vi "CRYO_MASTER_FULL_IP.vi"() -> ()   [LabVIEW 2017] (continued)
                n325 = invoke class="TabCtl (strict)" method="Get Image"(error in=errorcluster {"status"=FALSE, "code"=0, "source"=""} ("error in (no error)")) -> (error out=w580:errorcluster, "image data"=w582:T14)  [unwired: 5 in, 4 out]
                n326 = Build Path(base path=w591, name or relative path=w584) -> (appended path=w583:path)
                n327 = call <vilib>:"Write PNG File.vi"("error in (no error)"=w580, "image data"=w582, "path to PNG file"=w583) -> ("error out"=w578:errorcluster)  [unwired: 7 in, 1 out]
              }
            }
          }
          frame #1 {
            n328 = flat-sequence {
              tunnel: w595 -> [w598]
              tunnel: [w598] -> w594
              tunnel: w596 -> [w613]
              tunnel: w594 -> [w601]
              tunnel: [w600] -> w593
              tunnel: w592 -> [w599]
              frame #0 {
                n329 = property class="TabCtl (strict)"("Val(Sgnl)"=T2."LSI CONFIG" ("Value (Signaling)")) -> ()  [unwired: 2 in, 2 out]
              }
              frame #1 {
                w611 = "_" ("string")
                n330 = local read "Cycle #"() -> (w609:u32)
                n331 = call "LV_UNIXTIME.vi"("current time"=w601) -> ("date/time string"=w612:string)  [unwired: 9 in, 1 out]
                n332 = Format Value(format string="%06d", value (0)=w609) -> (output string=w608:string)  [unwired: 1 in]
                n333 = Concatenate Strings(w599, w612, w611, w608, w611, "page2.png" ("string")) -> (w606:string)
                n334 = invoke class="TabCtl (strict)" method="Get Image"(error in=errorcluster {"status"=FALSE, "code"=0, "source"=""} ("error in (no error)")) -> (error out=w602:errorcluster, "image data"=w604:T14)  [unwired: 5 in, 4 out]
                n335 = Build Path(base path=w613, name or relative path=w606) -> (appended path=w605:path)
                n336 = call <vilib>:"Write PNG File.vi"("error in (no error)"=w602, "image data"=w604, "path to PNG file"=w605) -> ("error out"=w600:errorcluster)  [unwired: 7 in, 1 out]
              }
            }
            n337 = local write "error out (frontpanel screenshots)"(w593) -> ()
          }
          frame #2 {
            n338 = flat-sequence {
              tunnel: w617 -> [w620]
              tunnel: [w620] -> w616
              tunnel: w618 -> [w635]
              tunnel: w616 -> [w623]
              tunnel: [w622] -> w615
              tunnel: w614 -> [w621]
              frame #0 {
                n339 = property class="TabCtl (strict)"("Val(Sgnl)"=T2."MEASUREMENT" ("Value (Signaling)")) -> ()  [unwired: 2 in, 2 out]
              }
              frame #1 {
                w633 = "_" ("string")
                n340 = local read "Cycle #"() -> (w631:u32)
                n341 = Format Value(format string="%06d", value (0)=w631) -> (output string=w630:string)  [unwired: 1 in]
                n342 = call "LV_UNIXTIME.vi"("current time"=w623) -> ("date/time string"=w634:string)  [unwired: 9 in, 1 out]
                n343 = Concatenate Strings(w621, w634, w633, w630, w633, "page3.png" ("string")) -> (w628:string)
                n344 = invoke class="TabCtl (strict)" method="Get Image"(error in=errorcluster {"status"=FALSE, "code"=0, "source"=""} ("error in (no error)")) -> (error out=w624:errorcluster, "image data"=w626:T14)  [unwired: 5 in, 4 out]
                n345 = Build Path(base path=w635, name or relative path=w628) -> (appended path=w627:path)
                n346 = call <vilib>:"Write PNG File.vi"("error in (no error)"=w624, "image data"=w626, "path to PNG file"=w627) -> ("error out"=w622:errorcluster)  [unwired: 7 in, 1 out]
              }
            }
            n347 = local write "error out (frontpanel screenshots)"(w615) -> ()
          }
          frame #3 {
            n348 = flat-sequence {
              tunnel: w639 -> [w642]
              tunnel: [w642] -> w638
              tunnel: w640 -> [w657]
              tunnel: w638 -> [w645]
              tunnel: [w644] -> w637
              tunnel: w636 -> [w643]
              frame #0 {
                n349 = property class="TabCtl (strict)"("Val(Sgnl)"=T2."HE AUTO FILL" ("Value (Signaling)")) -> ()  [unwired: 2 in, 2 out]
              }
              frame #1 {
                w655 = "_" ("string")
                n350 = local read "Cycle #"() -> (w653:u32)
                n351 = Format Value(format string="%06d", value (0)=w653) -> (output string=w652:string)  [unwired: 1 in]
                n352 = call "LV_UNIXTIME.vi"("current time"=w645) -> ("date/time string"=w656:string)  [unwired: 9 in, 1 out]
                n353 = Concatenate Strings(w643, w656, w655, w652, w655, "page4.png" ("string")) -> (w650:string)
                n354 = invoke class="TabCtl (strict)" method="Get Image"(error in=errorcluster {"status"=FALSE, "code"=0, "source"=""} ("error in (no error)")) -> (error out=w646:errorcluster, "image data"=w648:T14)  [unwired: 5 in, 4 out]
                n355 = Build Path(base path=w657, name or relative path=w650) -> (appended path=w649:path)
                n356 = call <vilib>:"Write PNG File.vi"("error in (no error)"=w646, "image data"=w648, "path to PNG file"=w649) -> ("error out"=w644:errorcluster)  [unwired: 7 in, 1 out]
              }
            }
            n357 = local write "error out (frontpanel screenshots)"(w637) -> ()
          }
          frame #4 {
            n358 = flat-sequence {
              tunnel: w661 -> [w664]
              tunnel: [w664] -> w660
              tunnel: w662 -> [w679]
              tunnel: w660 -> [w667]
              tunnel: [w666] -> w659
              tunnel: w658 -> [w665]
              frame #0 {
                n359 = property class="TabCtl (strict)"("Val(Sgnl)"=T2."VALVE/HEATER CTRL" ("Value (Signaling)")) -> ()  [unwired: 2 in, 2 out]
              }
              frame #1 {
                w677 = "_" ("string")
                n360 = local read "Cycle #"() -> (w675:u32)
                n361 = call "LV_UNIXTIME.vi"("current time"=w667) -> ("date/time string"=w678:string)  [unwired: 9 in, 1 out]
                n362 = Format Value(format string="%06d", value (0)=w675) -> (output string=w674:string)  [unwired: 1 in]
                n363 = Concatenate Strings(w665, w678, w677, w674, w677, "page5.png" ("string")) -> (w672:string)
                n364 = invoke class="TabCtl (strict)" method="Get Image"(error in=errorcluster {"status"=FALSE, "code"=0, "source"=""} ("error in (no error)")) -> (error out=w668:errorcluster, "image data"=w670:T14)  [unwired: 5 in, 4 out]
                n365 = Build Path(base path=w679, name or relative path=w672) -> (appended path=w671:path)
                n366 = call <vilib>:"Write PNG File.vi"("error in (no error)"=w668, "image data"=w670, "path to PNG file"=w671) -> ("error out"=w666:errorcluster)  [unwired: 7 in, 1 out]
              }
            }
            n367 = local write "error out (frontpanel screenshots)"(w659) -> ()
          }
          frame #5 {
            n368 = flat-sequence {
              tunnel: w683 -> [w686]
              tunnel: [w686] -> w682
              tunnel: w684 -> [w701]
              tunnel: w682 -> [w689]
              tunnel: [w688] -> w681
              tunnel: w680 -> [w687]
              frame #0 {
                n369 = property class="TabCtl (strict)"("Val(Sgnl)"=T2."DMMs" ("Value (Signaling)")) -> ()  [unwired: 2 in, 2 out]
              }
              frame #1 {
                w699 = "_" ("string")
                n370 = local read "Cycle #"() -> (w697:u32)
                n371 = call "LV_UNIXTIME.vi"("current time"=w689) -> ("date/time string"=w700:string)  [unwired: 9 in, 1 out]
                n372 = Format Value(format string="%06d", value (0)=w697) -> (output string=w696:string)  [unwired: 1 in]
                n373 = Concatenate Strings(w687, w700, w699, w696, w699, "page6.png" ("string")) -> (w694:string)
                n374 = invoke class="TabCtl (strict)" method="Get Image"(error in=errorcluster {"status"=FALSE, "code"=0, "source"=""} ("error in (no error)")) -> (error out=w690:errorcluster, "image data"=w692:T14)  [unwired: 5 in, 4 out]
                n375 = Build Path(base path=w701, name or relative path=w694) -> (appended path=w693:path)
                n376 = call <vilib>:"Write PNG File.vi"("error in (no error)"=w690, "image data"=w692, "path to PNG file"=w693) -> ("error out"=w688:errorcluster)  [unwired: 7 in, 1 out]
              }
            }
            n377 = local write "error out (frontpanel screenshots)"(w681) -> ()
          }
          frame #6 {
            n378 = flat-sequence {
              tunnel: w705 -> [w708]
              tunnel: [w708] -> w704
              tunnel: w706 -> [w723]
              tunnel: w704 -> [w711]
              tunnel: [w710] -> w703
              tunnel: w702 -> [w709]
              frame #0 {
                n379 = property class="TabCtl (strict)"("Val(Sgnl)"=T2."DIAGRAM" ("Value (Signaling)")) -> ()  [unwired: 2 in, 2 out]
              }
              frame #1 {
                w721 = "_" ("string")
                n380 = local read "Cycle #"() -> (w719:u32)
                n381 = Format Value(format string="%06d", value (0)=w719) -> (output string=w718:string)  [unwired: 1 in]
                n382 = call "LV_UNIXTIME.vi"("current time"=w711) -> ("date/time string"=w722:string)  [unwired: 9 in, 1 out]
                n383 = Concatenate Strings(w709, w722, w721, w718, w721, "page7.png" ("string")) -> (w716:string)
                n384 = invoke class="TabCtl (strict)" method="Get Image"(error in=errorcluster {"status"=FALSE, "code"=0, "source"=""} ("error in (no error)")) -> (error out=w712:errorcluster, "image data"=w714:T14)  [unwired: 5 in, 4 out]
                n385 = Build Path(base path=w723, name or relative path=w716) -> (appended path=w715:path)
                n386 = call <vilib>:"Write PNG File.vi"("error in (no error)"=w712, "image data"=w714, "path to PNG file"=w715) -> ("error out"=w710:errorcluster)  [unwired: 7 in, 1 out]
              }
            }
            n387 = local write "error out (frontpanel screenshots)"(w703) -> ()
          }
          frame #7 {
            n388 = flat-sequence {
              tunnel: w727 -> [w730]
              tunnel: [w730] -> w726
              tunnel: w728 -> [w745]
              tunnel: w726 -> [w733]
              tunnel: [w732] -> w725
              tunnel: w724 -> [w731]
              frame #0 {
                n389 = property class="TabCtl (strict)"("Val(Sgnl)"=T2."(Plc. hld.)" ("Value (Signaling)")) -> ()  [unwired: 2 in, 2 out]
              }
              frame #1 {
                w743 = "_" ("string")
                n390 = local read "Cycle #"() -> (w741:u32)
                n391 = Format Value(format string="%06d", value (0)=w741) -> (output string=w740:string)  [unwired: 1 in]
                n392 = call "LV_UNIXTIME.vi"("current time"=w733) -> ("date/time string"=w744:string)  [unwired: 9 in, 1 out]
                n393 = Concatenate Strings(w731, w744, w743, w740, w743, "page8.png" ("string")) -> (w738:string)
                n394 = invoke class="TabCtl (strict)" method="Get Image"(error in=errorcluster {"status"=FALSE, "code"=0, "source"=""} ("error in (no error)")) -> (error out=w734:errorcluster, "image data"=w736:T14)  [unwired: 5 in, 4 out]
                n395 = Build Path(base path=w745, name or relative path=w738) -> (appended path=w737:path)
                n396 = call <vilib>:"Write PNG File.vi"("error in (no error)"=w734, "image data"=w736, "path to PNG file"=w737) -> ("error out"=w732:errorcluster)  [unwired: 7 in, 1 out]
              }
            }
            n397 = local write "error out (frontpanel screenshots)"(w725) -> ()
          }
          frame #8 {
            n398 = local write "Frontpanel screenshots"(FALSE ("Frontpanel screenshots")) -> ()
          }
        }
        "error out (frontpanel screenshots)" <- w566
        n399 = property class="TabCtl (strict)"("Val(Sgnl)"=w564) -> ()  [unwired: 2 in, 2 out]
      }
      event "Stop Button": Value Change {
        n400 = event-data() -> ()  [unwired: 1 in, 3 out]
      }
    }
    n401 = Wait (ms)(milliseconds to wait=u32 123) -> ()  [unwired: 1 out]
  }
  n402 = while {
    stop <- w748 stop-if-true
    n403 = Wait (ms)(milliseconds to wait=u32 101) -> ()  [unwired: 1 out]
    n404 = event shown="[2] Timeout" {
      selector: _ -> [_ _ _]
      dyn-events: _ -> [_ _ _]
      timeout: _ -> [_ _ _]
      tunnel: [FALSE TRUE FALSE] -> w748
      event "Initialize (DMMs)": Value Change {
        w751 = T1 [] ("Value (Signaling)")
        n405 = event-data() -> ()  [unwired: 1 in, 3 out]
        n406 = property on="Graph DMMs 1" class="XYGraph (strict)"("Val(Sgnl)"=w751) -> ()  [unwired: 2 in, 2 out]
        n407 = property on="Graph DMMs 2" class="XYGraph (strict)"("Val(Sgnl)"=w751) -> ()  [unwired: 2 in, 2 out]
      }
      event "Stop Button": Value Change {
        n408 = event-data() -> ()  [unwired: 1 in, 3 out]
      }
      event Timeout {
        n409 = event-data() -> ()  [unwired: 1 in, 3 out]
      }
    }
  }
  n410 = Obtain Notifier(name (unnamed)="stop notifier", notification data type=w9, create if not found? (T)=w9, error in (no error)=errorcluster {"status"=FALSE, "code"=0, "source"=""}) -> (notifier out=w3:refnum<notifier>, error out=w2:errorcluster)  [unwired: 1 out]
  n411 = while {
    shift-right: [w852] -> w36
    shift-left: refnum<class "USBData.lvclass"> refnum ("USBData.lvclass") -> [w855]
    shift-right: [w848] -> w35
    shift-left: errorcluster {"status"=FALSE, "code"=0, "source"=""} ("error in (no error)") -> [w854]
    tunnel: "RUN label" -> [w760]
    tunnel: "Base Path" -> [w792]
    shift-right: [w830] -> w29
    shift-left: errorcluster {"status"=FALSE, "code"=0, "source"=""} ("error in (no error)") -> [w846]
    shift-right: [w831] -> w30
    shift-left: refnum<class "LSI218Data.lvclass"> refnum ("LSI218Data.lvclass") -> [w845]
    shift-right: [w818] -> w26
    shift-left: refnum<class "LSI336Data.lvclass"> refnum ("LSI336Data.lvclass") -> [w827]
    shift-right: [w817] -> w25
    shift-left: w15 -> [w826]
    shift-right: [w806] -> _
    shift-left: errorcluster {"status"=FALSE, "code"=0, "source"=""} ("error in") -> [w807]
    shift-right: [w796] -> w19
    shift-left: refnum<class "USBData.lvclass"> refnum ("USBData.lvclass") -> [w804]
    shift-right: [w795] -> w18
    shift-left: errorcluster {"status"=FALSE, "code"=0, "source"=""} ("error in (no error)") -> [w803]
    shift-right: [w791] -> _
    shift-left: w15 -> [w790]
    tunnel: w3 -> [w758]
    tunnel: w2 -> [w757]
    tunnel: [w755] -> w5
    tunnel: [w754] -> w4
    i -> [w767]
    stop <- "Stop Button" stop-if-true
    w813 = u32 24 ("Number of Rows")
    w823 = T20 [] ("appended array")
    w840 = T20 [] ("appended array")
    n412 = local read "LSI218Settings(A-F)"() -> (w782:T4)
    n413 = control-ref of="Plot selecter LSI218(2)\n    1      2     3     4"() -> (w811:refnum<vi>)
    n414 = control-ref of="Plot selecter LSI218(1)\n    1      2     3     4"() -> (w812:refnum<vi>)
    n415 = control-ref of="Plot selecter LSI336 \n     1      2     3     4"() -> (w810:refnum<vi>)
    n416 = property on="Property Node" class="Arr (strict)"(reference=w811, "Number of Rows"=w813) -> ()  [unwired: 1 in, 2 out]
    n417 = property on="Property Node" class="Arr (strict)"(reference=w812, "Number of Rows"=w813) -> ()  [unwired: 1 in, 2 out]
    n418 = local read "LSI336Settings(X,Y)"() -> (w780:T4)
    n419 = Array Size(array=w782) -> (size(s)=w781:i32)
    n420 = property on="Property Node" class="Arr (strict)"(reference=w810, "Number of Rows"=u32 8) -> ()  [unwired: 1 in, 2 out]
    n421 = Multiply(x="Measurement Interval (s)", y=u32 1000) -> (x*y=w849:dbl)
    n422 = Wait (ms)(milliseconds to wait=w849) -> ()  [unwired: 1 out]
    n423 = for {
      N: w781 -> [_]
      tunnel: w782 -> [w866] mode=indexing
      tunnel: [w865] -> w778 mode=concatenating
      n424 = Unbundle By Name(w866) -> ("SensorLocations"=w865:T13)
    }
    n425 = for {
      tunnel: w780 -> [w864] mode=indexing
      tunnel: [w863] -> w779 mode=concatenating
      n426 = Unbundle By Name(w864) -> ("SensorLocations"=w863:T13)
    }
    n427 = Quotient & Remainder(x=w767, y="Screenshots interval") -> (x-y*floor(x/y)=w765:i64)  [unwired: 1 out]
    n428 = Equal?(x=w767, y=0) -> (x = y?=w759:bool)
    n429 = case shown="True" w759 {
      tunnel: w855 -> [w1904 w1927]
      tunnel: w854 -> [w1898 w1925]
      tunnel: w767 -> [w1889 _]
      tunnel: [w1896 w1922] -> w848
      tunnel: [w1893 w1921] -> w805
      tunnel: [w1894 w1920] -> w852
      tunnel: [w1884 w1915] -> w853
      tunnel: w792 -> [_ w1914]
      tunnel: [w1883 w1911] -> w787
      frame False {
        n430 = call-dynamic "USBData_measure.vi"("USBData in"=w1904, "DAQ sample #"=i64 5, "DAQ timeout"=100.0 ("DAQ timeout (def: 100)"), "MeasurementIndex"=w1889, "error in (no error)"=w1898, "save every ... measurements"="Record interval") -> ("USBData out"=w1903:refnum<class "USBData.lvclass">, "TimeMeasuremeent"=w1900:timestamp, "Status"=→"USB6210 Status":T6, "LastDataAcquired"=w1885:dbl[], "error out"=w1899:errorcluster)  [unwired: 3 in, 2 out]
        "Time of Last Measurement (USB6210)" <- w1900
        "Last Vol\n(USB6210)" <- w1885
        n431 = call-dynamic "USBData_convert.vi"("Save every ... measurements"="Record interval", "MeasurementIndex"=w1889, "error in (no error)"=w1899, "LastDataAcquired"=w1885, "TimeMeasuremeent"=w1900, "USBData in"=w1903) -> ("error out"=w1897:errorcluster, "LeakDet_FULL"=w1892:dbl, "LastDataConverted"=w1886:dbl[], "USBData out"=w1895:refnum<class "USBData.lvclass">)  [unwired: 2 in]
        n432 = call "USBData_read.vi"("USBData in"=w1895, "error in (no error)"=w1897) -> ("Status"=w1887:T6, "USBData out"=w1894:refnum<class "USBData.lvclass">, "Data"=w1893:T21, "Basic"=w1884:T22, "error out"=w1896:errorcluster)  [unwired: 2 in, 2 out]
        n433 = local write "USB6210 Status"(w1887) -> ()
        n434 = Unbundle By Name(w1884) -> ("ReadLeakDet?"=w1891:bool)
        n435 = Unbundle By Name(w1884) -> ("Labels"=w1883:string[])
        n436 = case shown="False" w1891 {
          tunnel: w1886 -> [w1905 w1908]
          tunnel: w1892 -> [_ w1907]
          tunnel: [w1905 w1906] -> w1890
          frame False {
          }
          frame True {
            n437 = Build Array (concatenate)(w1908, w1907) -> (w1906:dbl[])
          }
        }
        "Last Data \n(USB6210)" <- w1890
      }
      frame True {
        n438 = local read "RUN Identifier"() -> (w1909:string)
        n439 = call-dynamic "USBData_initialize.vi"("USBData in"=w1927, "SeriesSetting"="USB6210 Config", "BasePath"=w1914, "RunIdentifier"=w1909, "FileName"="InstName (USB6210)", "error in (no error)"=w1925) -> ("Status"=w1910:T6, "USBData out"=w1923:refnum<class "USBData.lvclass">, "error out"=w1924:errorcluster)  [unwired: 5 in, 2 out]
        n440 = local write "USB6210 Status"(w1910) -> ()
        n441 = call "USBData_read.vi"("USBData in"=w1923, "error in (no error)"=w1924) -> ("Status"=w1913:T6, "USBData out"=w1920:refnum<class "USBData.lvclass">, "Data"=w1921:T21, "Basic"=w1915:T22, "error out"=w1922:errorcluster)  [unwired: 2 in, 2 out]
        n442 = local write "USB6210 Status"(w1913) -> ()
        n443 = Unbundle By Name(w1915) -> ("ReadLeakDet?"=w1919:bool, "Labels"=w1911:string[])
        n444 = Array Size(array=w1911) -> (size(s)=w1918:i32)
        n445 = case shown="True" w1919 {
          tunnel: w1918 -> [w1928 w1930]
          tunnel: [w1928 w1929] -> w1916
          frame False {
          }
          frame True {
            n446 = Add(x=w1930, y=1) -> (x+y=w1929:i32)
          }
        }
        n447 = Initialize Array(TRUE ("Activate 2"), w1916) -> ()  [unwired: 1 out]
      }
    }
    "error out (USB6210)" <- w848
    n448 = case shown="False" w759 {
      tunnel: [w1437 w1464] -> w795
      tunnel: [w1434 w1463] -> w802
      tunnel: [w1435 w1462] -> w796
      tunnel: [w1426 w1457] -> w801
      tunnel: [w1425 w1455] -> _
      tunnel: w804 -> [w1424 w1453]
      tunnel: w792 -> [_ w1452]
      tunnel: w803 -> [w1423 w1451]
      tunnel: w767 -> [w1422 _]
      frame False {
        n449 = local read "Record interval"() -> (w1421:i64)
        n450 = call-dynamic "USBData_measure.vi"("USBData in"=w1424, "DAQ sample #"=i64 5, "DAQ timeout"=100.0 ("DAQ timeout (def: 100)"), "MeasurementIndex"=w1422, "error in (no error)"=w1423, "save every ... measurements"=w1421) -> ("USBData out"=w1443:refnum<class "USBData.lvclass">, "TimeMeasuremeent"=w1440:timestamp, "Status"=→"USB6218 Status":T6, "LastDataAcquired"=w1427:dbl[], "error out"=w1439:errorcluster)  [unwired: 3 in, 2 out]
        "Time of Last Measurement (USB6218)" <- w1440
        "Last Vol \n(USB6218)" <- w1427
        n451 = call-dynamic "USBData_convert.vi"("Save every ... measurements"=w1421, "MeasurementIndex"=w1422, "error in (no error)"=w1439, "LastDataAcquired"=w1427, "TimeMeasuremeent"=w1440, "USBData in"=w1443) -> ("error out"=w1438:errorcluster, "LeakDet_FULL"=w1433:dbl, "LastDataConverted"=w1428:dbl[], "USBData out"=w1436:refnum<class "USBData.lvclass">)  [unwired: 2 in]
        n452 = call "USBData_read.vi"("USBData in"=w1436, "error in (no error)"=w1438) -> ("Status"=w1429:T6, "USBData out"=w1435:refnum<class "USBData.lvclass">, "Data"=w1434:T21, "Basic"=w1426:T22, "error out"=w1437:errorcluster)  [unwired: 2 in, 2 out]
        n453 = local write "USB6218 Status"(w1429) -> ()
        n454 = Unbundle By Name(w1426) -> ("ReadLeakDet?"=w1432:bool)
        n455 = Unbundle By Name(w1426) -> ("Labels"=w1425:string[])
        n456 = case shown="True" w1432 {
          tunnel: w1428 -> [w1444 w1447]
          tunnel: w1433 -> [_ w1446]
          tunnel: [w1444 w1445] -> w1431
          frame False {
          }
          frame True {
            n457 = Build Array (concatenate)(w1447, w1446) -> (w1445:dbl[])
          }
        }
        "Last Data \n(USB6218)" <- w1431
      }
      frame True {
        n458 = local read "RUN Identifier"() -> (w1448:string)
        n459 = call-dynamic "USBData_initialize.vi"("USBData in"=w1453, "SeriesSetting"="USB6218 Config", "BasePath"=w1452, "RunIdentifier"=w1448, "FileName"="InstName (USB6218)", "error in (no error)"=w1451) -> ("Status"=w1449:T6, "USBData out"=w1465:refnum<class "USBData.lvclass">, "error out"=w1466:errorcluster)  [unwired: 5 in, 2 out]
        n460 = local write "USB6218 Status"(w1449) -> ()
        n461 = call "USBData_read.vi"("USBData in"=w1465, "error in (no error)"=w1466) -> ("Status"=w1456:T6, "USBData out"=w1462:refnum<class "USBData.lvclass">, "Data"=w1463:T21, "Basic"=w1457:T22, "error out"=w1464:errorcluster)  [unwired: 2 in, 2 out]
        n462 = local write "USB6218 Status"(w1456) -> ()
        n463 = Unbundle By Name(w1457) -> ("ReadLeakDet?"=w1461:bool, "Labels"=w1455:string[])
        n464 = Array Size(array=w1455) -> (size(s)=w1460:i32)
        n465 = case shown="True" w1461 {
          tunnel: w1460 -> [w1467 w1469]
          tunnel: [w1467 w1468] -> w1458
          frame False {
          }
          frame True {
            n466 = Add(x=w1469, y=1) -> (x+y=w1468:i32)
          }
        }
        n467 = Initialize Array(TRUE ("Activate 2"), w1458) -> ()  [unwired: 1 out]
      }
    }
    "error out (USB6218)" <- w795
    n468 = case shown="True" w759 {
      tunnel: w760 -> [_ w858]
      frame False {
      }
      frame True {
        n469 = Get Date/Time In Seconds() -> (seconds since 1Jan1904=w861:timestamp)
        n470 = call "LV_UNIXTIME.vi"("current time"=w861) -> ("date/time string"=w860:string)  [unwired: 9 in, 1 out]
        n471 = Concatenate Strings(w860, "_" ("string"), w858) -> (→"RUN Identifier" →"RUN Identifier 2" →"RUN Identifier 3" →"RUN Identifier 4" →"RUN Identifier 5" →"RUN Identifier 6" →"RUN Identifier 7":string)
      }
    }
    n472 = Equal?(x=w765, y=i64 0) -> (x = y?=w762:bool)
    n473 = local read "LastData (LSI218)"() -> (w776:dbl[])
    n474 = local read "Last Data \nLSI336"() -> (w775:dbl[])
    n475 = And(x="Analog Out ON?", y=w759) -> (x .and. y?=w793:bool)
    n476 = case shown="True" w793 {
      tunnel: w792 -> [_ w1238]
      tunnel: [w1221 w1229] -> w791
      tunnel: w790 -> [w1221 w1228]
      frame False {
      }
      frame True {
        w1224 = "_raw" ("string")
        w1245 = 10.0 ("V_lim_max")
        w1244 = 0.0 ("V_lim_min")
        w1243 = -1 items=["Default"=-1, "RSE"=10083, "Differential"=10106, "Pseudodifferential"=12529] ("output terminal configuration")
        w1242 = 10348 items=["Volts"=10348, "From Custom Scale"=10065] ("units")
        n477 = local read "RUN Identifier"() -> (w1222:string)
        n478 = Concatenate Strings(w1222, "_AO" ("string")) -> (w1247:string)
        n479 = Concatenate Strings(w1222, "_", "USB_AOUT.csv" ("string")) -> (w1239:string)
        n480 = Build Path(base path=w1238, name or relative path=w1239) -> (appended path=w1235:path)
        n481 = Concatenate Strings("AOUT 0 Label", w1224) -> (w1226:string)
        n482 = Concatenate Strings("AOUT 1 Label", w1224) -> (w1223:string)
        n483 = Open/Create/Replace File(file path (use dialog)=w1235, operation (0:open)=T19."open or create") -> (refnum out=w1233:refnum<file>)  [unwired: 4 in, 2 out]
        n484 = Build Array("AOUT 0 Label", "AOUT 1 Label", w1226, w1223) -> (w1231:string[])
        n485 = call "FileIntialize.vi"("Error In"=w1228, "Labels"=w1231, "refnum in"=w1233) -> ("Error Out"=w1230:errorcluster, "File Refnum"=→"File Refn USB AO":refnum<file>)  [unwired: 7 in]
        n486 = call <vilib>:"DAQmx Create Task.vi"("new task name"=w1247, "auto cleanup"=FALSE, "error in"=w1230) -> ("task out"=w1246:refnum<k21>, "error out"=w1248:errorcluster)  [unwired: 11 in]
        n487 = call-poly <vilib>:"DAQmx Create Virtual Channel.vi"("task in"=w1246, "maximum value"=w1245, "minimum value"=w1244, "output terminal configuration"=w1243, "physical channels"="AOUT For Voltage CTRL", "units"=w1242, "error in"=w1248) -> ("task out"=w1250:refnum<k21>, "error out"=w1251:errorcluster)  [unwired: 7 in]
        n488 = call-poly <vilib>:"DAQmx Create Virtual Channel.vi"("task in"=w1250, "maximum value"=w1245, "minimum value"=w1244, "physical channels"="AOUT for Current CTRL", "error in"=w1251) -> ("task out"=w1253:refnum<k21>, "error out"=w1252:errorcluster)  [unwired: 9 in]
        n489 = call <vilib>:"DAQmx Start Task.vi"("task/channels in"=w1253, "error in"=w1252) -> ("task out"=→"AO task out":refnum<k21>, "error out"=w1229:errorcluster)  [unwired: 12 in]
      }
    }
    "error out (USB6210/6218 AOUT)" <- w791
    n490 = And(x=w762, y="Automatic \nScreenshots?") -> (x .and. y?=w761:bool)
    n491 = Build Array (concatenate)(w776, w775) -> (w774:dbl[])
    "AllTemperatures" <- w774
    n492 = Build Array (concatenate)(w778, w779) -> (w777:T13)
    "TempSensorsLocations" <- w777
    n493 = case shown="True" w761 {
      frame False {
      }
      frame True {
        n494 = flat-sequence {
          frame #0 {
            n495 = property on="Frontpanel screenshots" class="Bool (strict)"("Val(Sgnl)"=TRUE ("Value (Signaling)")) -> ()  [unwired: 2 in, 2 out]
          }
        }
      }
    }
    n496 = flat-sequence {
      tunnel: w774 -> [w867]
      tunnel: w777 -> [w868]
      tunnel: w769 -> [w1120]
      tunnel: w768 -> [w1119]
      frame #0 {
        n497 = stacked-sequence {
          tunnel: w868 -> [w873 w878 w883 w888 w893 w898 w903 w908 w913 w918 w923 w928 w933 w938 w943 w948 w953 w958 w963 w968 w973 w978 w983 w988 w993 w998 w1003 w1008 w1013 w1018 w1023 w1028 w1033 w1038 w1043 w1048 w1053 w1058 w1063 w1068 w1073 w1078 w1083 w1088 w1093 w1098 w1103 w1108 w1113 w1118]
          tunnel: w867 -> [w871 w876 w881 w886 w891 w896 w901 w906 w911 w916 w921 w926 w931 w936 w941 w946 w951 w956 w961 w966 w971 w976 w981 w986 w991 w996 w1001 w1006 w1011 w1016 w1021 w1026 w1031 w1036 w1041 w1046 w1051 w1056 w1061 w1066 w1071 w1076 w1081 w1086 w1091 w1096 w1101 w1106 w1111 w1116]
          frame #0 {
            n498 = Search 1D Array(1D array=w873, element=T11."T3He1-1" ("SensorLocations")) -> (index of element=w870:i32)  [unwired: 1 in]
            n499 = Index Array(array=w871, index=w870) -> (element=→"T3He1-1":dbl)
          }
          frame #1 {
            n500 = Search 1D Array(1D array=w878, element=T11."T3He1-2" ("SensorLocations")) -> (index of element=w875:i32)  [unwired: 1 in]
            n501 = Index Array(array=w876, index=w875) -> (element=→"T3He1-2":dbl)
          }
          frame #2 {
            n502 = Search 1D Array(1D array=w883, element=T11."T3He1-3" ("SensorLocations")) -> (index of element=w880:i32)  [unwired: 1 in]
            n503 = Index Array(array=w881, index=w880) -> (element=→"T3He1-3":dbl)
          }
          frame #3 {
            n504 = Search 1D Array(1D array=w888, element=T11."T3He1-4" ("SensorLocations")) -> (index of element=w885:i32)  [unwired: 1 in]
            n505 = Index Array(array=w886, index=w885) -> (element=→"T3He1-4":dbl)
          }
          frame #4 {
            n506 = Search 1D Array(1D array=w893, element=T11."T3He2-1" ("SensorLocations")) -> (index of element=w890:i32)  [unwired: 1 in]
            n507 = Index Array(array=w891, index=w890) -> (element=→"T3He2-1":dbl)
          }
          frame #5 {
            n508 = Search 1D Array(1D array=w898, element=T11."T3He2-2" ("SensorLocations")) -> (index of element=w895:i32)  [unwired: 1 in]
            n509 = Index Array(array=w896, index=w895) -> (element=→"T3He2-2":dbl)
          }
          frame #6 {
            n510 = Search 1D Array(1D array=w903, element=T11."T3He3" ("SensorLocations")) -> (index of element=w900:i32)  [unwired: 1 in]
            n511 = Index Array(array=w901, index=w900) -> (element=→"T3He3":dbl)
          }
          frame #7 {
            n512 = Search 1D Array(1D array=w908, element=T11."T3He4" ("SensorLocations")) -> (index of element=w905:i32)  [unwired: 1 in]
            n513 = Index Array(array=w906, index=w905) -> (element=→"T3He4":dbl)
          }
          frame #8 {
            n514 = Search 1D Array(1D array=w913, element=T11."T3He5" ("SensorLocations")) -> (index of element=w910:i32)  [unwired: 1 in]
            n515 = Index Array(array=w911, index=w910) -> (element=→"T3He5":dbl)
          }
          frame #9 {
            n516 = Search 1D Array(1D array=w918, element=T11."T3He6-1" ("SensorLocations")) -> (index of element=w915:i32)  [unwired: 1 in]
            n517 = Index Array(array=w916, index=w915) -> (element=→"T3He6-1" →"T3He6-1/6-2 (HEX1)":dbl)
          }
          frame #10 {
            n518 = Search 1D Array(1D array=w923, element=T11."T3He6-2" ("SensorLocations")) -> (index of element=w920:i32)  [unwired: 1 in]
            n519 = Index Array(array=w921, index=w920) -> (element=→"T3He6-2" →"T3He6-1/6-2 (3He pot) 2":dbl)
          }
          frame #11 {
            n520 = Search 1D Array(1D array=w928, element=T11."T3He7-1" ("SensorLocations")) -> (index of element=w925:i32)  [unwired: 1 in]
            n521 = Index Array(array=w926, index=w925) -> (element=→"T3He7-1" →"T3He7-1/7-2 (HEX1)":dbl)
          }
          frame #12 {
            n522 = Search 1D Array(1D array=w933, element=T11."T3He7-2" ("SensorLocations")) -> (index of element=w930:i32)  [unwired: 1 in]
            n523 = Index Array(array=w931, index=w930) -> (element=→"T3He7-2" →"T3He7-1/6-2 (3He pot) 2":dbl)
          }
          frame #13 {
            n524 = Search 1D Array(1D array=w938, element=T11."T3He8" ("SensorLocations")) -> (index of element=w935:i32)  [unwired: 1 in]
            n525 = Index Array(array=w936, index=w935) -> (element=→"T3He8":dbl)
          }
          frame #14 {
            n526 = Search 1D Array(1D array=w943, element=T11."T3He9" ("SensorLocations")) -> (index of element=w940:i32)  [unwired: 1 in]
            n527 = Index Array(array=w941, index=w940) -> (element=→"T3He9":dbl)
          }
          frame #15 {
            n528 = Search 1D Array(1D array=w948, element=T11."T3He10" ("SensorLocations")) -> (index of element=w945:i32)  [unwired: 1 in]
            n529 = Index Array(array=w946, index=w945) -> (element=→"T3He10":dbl)
          }
          frame #16 {
            n530 = Search 1D Array(1D array=w953, element=T11."T4He1" ("SensorLocations")) -> (index of element=w950:i32)  [unwired: 1 in]
            n531 = Index Array(array=w951, index=w950) -> (element=→"T4He1" →"T4He1 (4K reservoir )":dbl)
          }
          frame #17 {
            n532 = Search 1D Array(1D array=w958, element=T11."T4He2-1" ("SensorLocations")) -> (index of element=w955:i32)  [unwired: 1 in]
            n533 = Index Array(array=w956, index=w955) -> (element=→"T4He2-1":dbl)
          }
          frame #18 {
            n534 = Search 1D Array(1D array=w963, element=T11."T4He2-2" ("SensorLocations")) -> (index of element=w960:i32)  [unwired: 1 in]
            n535 = Index Array(array=w961, index=w960) -> (element=→"T4He2-2":dbl)
          }
          frame #19 {
            n536 = Search 1D Array(1D array=w968, element=T11."T4He3-1" ("SensorLocations")) -> (index of element=w965:i32)  [unwired: 1 in]
            n537 = Index Array(array=w966, index=w965) -> (element=→"T4He3-1":dbl)
          }
          frame #20 {
            n538 = Search 1D Array(1D array=w973, element=T11."T4He3-2" ("SensorLocations")) -> (index of element=w970:i32)  [unwired: 1 in]
            n539 = Index Array(array=w971, index=w970) -> (element=→"T4He3-2":dbl)
          }
          frame #21 {
            n540 = Search 1D Array(1D array=w978, element=T11."T4He3-3" ("SensorLocations")) -> (index of element=w975:i32)  [unwired: 1 in]
            n541 = Index Array(array=w976, index=w975) -> (element=→"T4He3-3":dbl)
          }
          frame #22 {
            n542 = Search 1D Array(1D array=w983, element=T11."T4He3-4" ("SensorLocations")) -> (index of element=w980:i32)  [unwired: 1 in]
            n543 = Index Array(array=w981, index=w980) -> (element=→"T4He3-4":dbl)
          }
          frame #23 {
            n544 = Search 1D Array(1D array=w988, element=T11."T4He4" ("SensorLocations")) -> (index of element=w985:i32)  [unwired: 1 in]
            n545 = Index Array(array=w986, index=w985) -> (element=→"T4He4":dbl)
          }
          frame #24 {
            n546 = Search 1D Array(1D array=w993, element=T11."T4He5" ("SensorLocations")) -> (index of element=w990:i32)  [unwired: 1 in]
            n547 = Index Array(array=w991, index=w990) -> (element=→"T4He5":dbl)
          }
          frame #25 {
            n548 = Search 1D Array(1D array=w998, element=T11."T4He6" ("SensorLocations")) -> (index of element=w995:i32)  [unwired: 1 in]
            n549 = Index Array(array=w996, index=w995) -> (element=→"T4He6":dbl)
          }
          frame #26 {
            n550 = Search 1D Array(1D array=w1003, element=T11."T4He7" ("SensorLocations")) -> (index of element=w1000:i32)  [unwired: 1 in]
            n551 = Index Array(array=w1001, index=w1000) -> (element=→"T4He7":dbl)
          }
          frame #27 {
            n552 = Search 1D Array(1D array=w1008, element=T11."T4He8" ("SensorLocations")) -> (index of element=w1005:i32)  [unwired: 1 in]
            n553 = Index Array(array=w1006, index=w1005) -> (element=→"T4He8":dbl)
          }
          frame #28 {
            n554 = Search 1D Array(1D array=w1013, element=T11."T4He9" ("SensorLocations")) -> (index of element=w1010:i32)  [unwired: 1 in]
            n555 = Index Array(array=w1011, index=w1010) -> (element=→"T4He9":dbl)
          }
          frame #29 {
            n556 = Search 1D Array(1D array=w1018, element=T11."T4He10" ("SensorLocations")) -> (index of element=w1015:i32)  [unwired: 1 in]
            n557 = Index Array(array=w1016, index=w1015) -> (element=→"T4He10":dbl)
          }
          frame #30 {
            n558 = Search 1D Array(1D array=w1023, element=T11."T1K1" ("SensorLocations")) -> (index of element=w1020:i32)  [unwired: 1 in]
            n559 = Index Array(array=w1021, index=w1020) -> (element=→"T1K1":dbl)
          }
          frame #31 {
            n560 = Search 1D Array(1D array=w1028, element=T11."T1K2" ("SensorLocations")) -> (index of element=w1025:i32)  [unwired: 1 in]
            n561 = Index Array(array=w1026, index=w1025) -> (element=→"T1K2":dbl)
          }
          frame #32 {
            n562 = Search 1D Array(1D array=w1033, element=T11."T1K3-1" ("SensorLocations")) -> (index of element=w1030:i32)  [unwired: 1 in]
            n563 = Index Array(array=w1031, index=w1030) -> (element=→"T1K3-1" →"T1K3-1/3-2 (1K pot)":dbl)
          }
          frame #33 {
            n564 = Search 1D Array(1D array=w1038, element=T11."T1K3-2" ("SensorLocations")) -> (index of element=w1035:i32)  [unwired: 1 in]
            n565 = Index Array(array=w1036, index=w1035) -> (element=→"T1K3-2" →"T1K3-1/3-2 (1K pot) 2":dbl)
          }
          frame #34 {
            n566 = Search 1D Array(1D array=w1043, element=T11."T1K4" ("SensorLocations")) -> (index of element=w1040:i32)  [unwired: 1 in]
            n567 = Index Array(array=w1041, index=w1040) -> (element=→"T1K4":dbl)
          }
          frame #35 {
            n568 = Search 1D Array(1D array=w1048, element=T11."T1K5" ("SensorLocations")) -> (index of element=w1045:i32)  [unwired: 1 in]
            n569 = Index Array(array=w1046, index=w1045) -> (element=→"T1K5":dbl)
          }
          frame #36 {
            n570 = Search 1D Array(1D array=w1053, element=T11."T1K6" ("SensorLocations")) -> (index of element=w1050:i32)  [unwired: 1 in]
            n571 = Index Array(array=w1051, index=w1050) -> (element=→"T1K6":dbl)
          }
          frame #37 {
            n572 = Search 1D Array(1D array=w1058, element=T11."TIP1" ("SensorLocations")) -> (index of element=w1055:i32)  [unwired: 1 in]
            n573 = Index Array(array=w1056, index=w1055) -> (element=→"TIP1":dbl)
          }
          frame #38 {
            n574 = Search 1D Array(1D array=w1063, element=T11."TIP2" ("SensorLocations")) -> (index of element=w1060:i32)  [unwired: 1 in]
            n575 = Index Array(array=w1061, index=w1060) -> (element=→"TIP2":dbl)
          }
          frame #39 {
            n576 = Search 1D Array(1D array=w1068, element=T11."TIP3" ("SensorLocations")) -> (index of element=w1065:i32)  [unwired: 1 in]
            n577 = Index Array(array=w1066, index=w1065) -> (element=→"TIP3":dbl)
          }
          frame #40 {
            n578 = Search 1D Array(1D array=w1073, element=T11."TIP4" ("SensorLocations")) -> (index of element=w1070:i32)  [unwired: 1 in]
            n579 = Index Array(array=w1071, index=w1070) -> (element=→"TIP4":dbl)
          }
          frame #41 {
            n580 = Search 1D Array(1D array=w1078, element=T11."TIP5" ("SensorLocations")) -> (index of element=w1075:i32)  [unwired: 1 in]
            n581 = Index Array(array=w1076, index=w1075) -> (element=→"TIP5":dbl)
          }
          frame #42 {
            n582 = Search 1D Array(1D array=w1083, element=T11."TIP6" ("SensorLocations")) -> (index of element=w1080:i32)  [unwired: 1 in]
            n583 = Index Array(array=w1081, index=w1080) -> (element=→"TIP6":dbl)
          }
          frame #43 {
            n584 = Search 1D Array(1D array=w1088, element=T11."TIP7" ("SensorLocations")) -> (index of element=w1085:i32)  [unwired: 1 in]
            n585 = Index Array(array=w1086, index=w1085) -> (element=→"TIP7":dbl)
          }
          frame #44 {
            n586 = Search 1D Array(1D array=w1093, element=T11."TTH1" ("SensorLocations")) -> (index of element=w1090:i32)  [unwired: 1 in]
            n587 = Index Array(array=w1091, index=w1090) -> (element=→"TTH1":dbl)
          }
          frame #45 {
            n588 = Search 1D Array(1D array=w1098, element=T11."TTH2" ("SensorLocations")) -> (index of element=w1095:i32)  [unwired: 1 in]
            n589 = Index Array(array=w1096, index=w1095) -> (element=→"TTH2":dbl)
          }
          frame #46 {
            n590 = Search 1D Array(1D array=w1103, element=T11."TTH3" ("SensorLocations")) -> (index of element=w1100:i32)  [unwired: 1 in]
            n591 = Index Array(array=w1101, index=w1100) -> (element=→"TTH3":dbl)
          }
          frame #47 {
            n592 = Search 1D Array(1D array=w1108, element=T11."TTH4" ("SensorLocations")) -> (index of element=w1105:i32)  [unwired: 1 in]
            n593 = Index Array(array=w1106, index=w1105) -> (element=→"TTH4":dbl)
          }
          frame #48 {
            n594 = Search 1D Array(1D array=w1113, element="SensorLocation 1") -> (index of element=w1110:i32)  [unwired: 1 in]
            n595 = Index Array(array=w1111, index=w1110) -> (element=→"Temperature 1":dbl)
          }
          frame #49 {
            n596 = Search 1D Array(1D array=w1118, element="SensorLocation 2") -> (index of element=w1115:i32)  [unwired: 1 in]
            n597 = Index Array(array=w1116, index=w1115) -> (element=→"Temperature 2":dbl)
          }
        }
      }
      frame #1 {
        n598 = stacked-sequence {
          tunnel: w1120 -> [w1125 w1130 w1135 w1140 w1145 w1150 w1155 w1160 w1165 w1170 w1175 w1180 w1185 w1190 w1195 w1200 w1205 w1210 w1215 w1220]
          tunnel: w1119 -> [w1122 w1128 w1134 w1139 w1144 w1148 w1153 w1158 w1163 w1168 w1173 w1178 w1183 w1187 w1192 w1197 w1202 w1207 w1212 w1217]
          frame #0 {
            n599 = Search 1D Array(1D array=w1125, element="Insulation vacuum") -> (index of element=w1123:i32)  [unwired: 1 in]
            n600 = Index Array(array=w1122, index=w1123) -> (element=→"P_ins" →"P (insulation)":dbl)
          }
          frame #1 {
            n601 = Search 1D Array(1D array=w1130, element="4K reservoir pressure") -> (index of element=w1127:i32)  [unwired: 1 in]
            n602 = Index Array(array=w1128, index=w1127) -> (element=→"P_4Kres" →"P (4K reservoir)":dbl)
          }
          frame #2 {
            n603 = Search 1D Array(1D array=w1135, element="3He inlet pressure") -> (index of element=w1133:i32)  [unwired: 1 in]
            n604 = Index Array(array=w1134, index=w1133) -> (element=→"P_3HeIN" →"P (3He IN)":dbl)
          }
          frame #3 {
            n605 = Search 1D Array(1D array=w1140, element="Shield return press.") -> (index of element=w1138:i32)  [unwired: 1 in]
            n606 = Index Array(array=w1139, index=w1138) -> (element=→"P_SldRTN" →"P (shield return)":dbl)
          }
          frame #4 {
            n607 = Search 1D Array(1D array=w1145, element="3He pot pressure") -> (index of element=w1143:i32)  [unwired: 1 in]
            n608 = Index Array(array=w1144, index=w1143) -> (element=→"P_3Hepot" →"P (3He pot)":dbl)
          }
          frame #5 {
            n609 = Search 1D Array(1D array=w1150, element="1Kpot pressure") -> (index of element=w1147:i32)  [unwired: 1 in]
            n610 = Index Array(array=w1148, index=w1147) -> (element=→"P_1Kpot" →"P (1K pot)":dbl)
          }
          frame #6 {
            n611 = Search 1D Array(1D array=w1155, element="Dewar pressure") -> (index of element=w1152:i32)  [unwired: 1 in]
            n612 = Index Array(array=w1153, index=w1152) -> (element=→"P_Dewar" →"P (Dewar)":dbl)
          }
          frame #7 {
            n613 = Search 1D Array(1D array=w1160, element="HEX7 out pressure") -> (index of element=w1157:i32)  [unwired: 1 in]
            n614 = Index Array(array=w1158, index=w1157) -> (element=→"P_HEX7OUT" →"P (HEX7 out)":dbl)
          }
          frame #8 {
            n615 = Search 1D Array(1D array=w1165, element="IPHe pressure") -> (index of element=w1162:i32)  [unwired: 1 in]
            n616 = Index Array(array=w1163, index=w1162) -> (element=→"P_IPHe" →"P (IPHe)":dbl)
          }
          frame #9 {
            n617 = Search 1D Array(1D array=w1170, element="Diff pressure HEX4") -> (index of element=w1167:i32)  [unwired: 1 in]
            n618 = Index Array(array=w1168, index=w1167) -> (element=→"DP_HEX4" →"DP HEX4":dbl)
          }
          frame #10 {
            n619 = Search 1D Array(1D array=w1175, element="Diff pressure HEX5") -> (index of element=w1172:i32)  [unwired: 1 in]
            n620 = Index Array(array=w1173, index=w1172) -> (element=→"DP_HEX5" →"DP HEX5":dbl)
          }
          frame #11 {
            n621 = Search 1D Array(1D array=w1180, element="1K pump exhaust flow") -> (index of element=w1177:i32)  [unwired: 1 in]
            n622 = Index Array(array=w1178, index=w1177) -> (element=→"F_1" →"F1 (1K pump exhaust) flow":dbl)
          }
          frame #12 {
            n623 = Search 1D Array(1D array=w1185, element="Shield flow") -> (index of element=w1182:i32)  [unwired: 1 in]
            n624 = Index Array(array=w1183, index=w1182) -> (element=→"F_2" →"F2 (shield flow)":dbl)
          }
          frame #13 {
            n625 = Search 1D Array(1D array=w1190, element="4He return flow from HEX7") -> (index of element=w1188:i32)  [unwired: 1 in]
            n626 = Index Array(array=w1187, index=w1188) -> (element=→"F_3" →"F3 (4He rtn flw via HEX7)":dbl)
          }
          frame #14 {
            n627 = Search 1D Array(1D array=w1195, element="3He incoming flow into HEX7") -> (index of element=w1193:i32)  [unwired: 1 in]
            n628 = Index Array(array=w1192, index=w1193) -> (element=→"F_4" →"F4 (3He in to HEX7)":dbl)
          }
          frame #15 {
            n629 = Search 1D Array(1D array=w1200, element="3He pump exhaust flow") -> (index of element=w1198:i32)  [unwired: 1 in]
            n630 = Index Array(array=w1197, index=w1198) -> (element=→"F_5" →"F5 (3He pump ex.)":dbl)
          }
          frame #16 {
            n631 = Search 1D Array(1D array=w1205, element="4K reservoir level") -> (index of element=w1203:i32)  [unwired: 1 in]
            n632 = Index Array(array=w1202, index=w1203) -> (element=→"L3" →"He level (4K)":dbl)
          }
          frame #17 {
            n633 = Search 1D Array(1D array=w1210, element="1K pot level") -> (index of element=w1208:i32)  [unwired: 1 in]
            n634 = Index Array(array=w1207, index=w1208) -> (element=→"L(1K) (a1)" →"He level (1K)":dbl)
          }
          frame #18 {
            n635 = Search 1D Array(1D array=w1215, element="1K pot (b)") -> (index of element=w1213:i32)  [unwired: 1 in]
            n636 = Index Array(array=w1212, index=w1213) -> (element=→"1K pot(b1)" →"He level (1K) b":dbl)
          }
          frame #19 {
            n637 = Search 1D Array(1D array=w1220, element="3He pot") -> (index of element=w1218:i32)  [unwired: 1 in]
            n638 = Index Array(array=w1217, index=w1218) -> (element=→"3He pot level" →"He level (3He)":dbl)
          }
        }
      }
    }
    n639 = case shown="True" w759 {
      tunnel: [w1864 w1879] -> w830
      tunnel: [w1859 w1878] -> w847
      tunnel: [w1862 w1877] -> w831
      tunnel: w767 -> [w1863 _]
      tunnel: w846 -> [w1853 w1872]
      tunnel: w845 -> [w1854 w1871]
      tunnel: w792 -> [_ w1870]
      tunnel: [w1851 timestamp[] [] ("TimeArray")] -> w844
      tunnel: [w1850 dbl[][] [] ("DataArray")] -> w843
      frame False {
        w1857 = 24 ("index")
        n640 = local read "Record interval"() -> (w1848:i64)
        n641 = call-dynamic "LSI218Data_measure.vi"("LSI218Data in"=w1854, "MeasurementIndex"=w1863, "error in (no error)"=w1853, "save every ... measurements"=w1848) -> ("TimeMeasuremeent"=→"Time of Last Measurement (LSI218)":timestamp, "Active?"=w1858:bool[], "LSI218Data out"=w1862:refnum<class "LSI218Data.lvclass">, "LastMeasurementConfig"=→"LastMeasurementConfig (218)":T12, "LastData"=w1852:dbl[], "Status"=w1859:u16, "TimeArray"=w1851:timestamp[], "DataArray"=w1850:dbl[][], "error out"=w1864:errorcluster)  [unwired: 3 in]
        "LastData (LSI218)" <- w1852
        n642 = Split 1D Array(array=w1858, index=w1857) -> (first subarray=→"Active?\n (1)":bool[], second subarray=→"Active?\n(2)":bool[])
        n643 = Split 1D Array(array=w1852, index=w1857) -> (first subarray=→"Last Data \nLSI218 (1)":dbl[], second subarray=→"Last Data \nLSI218 (2)":dbl[])
      }
      frame True {
        n644 = local read "RUN Identifier"() -> (w1866:string)
        n645 = call-dynamic "LSI218Data_initialize.vi"("LSI218Settings(A-F)"="LSI218Settings(A-F)", "FileFormat"="FileFormat (218)", "base path"=w1870, "error in (no error)"=w1872, "InstName"="InstName (LSI218)", "RunIdentifier"=w1866, "LSI218Data in"=w1871) -> ("error out"=w1879:errorcluster, "Status"=w1878:T7, "AllLabels"=w1869:string[], "LSI218Data out"=w1877:refnum<class "LSI218Data.lvclass">)  [unwired: 1 in]
        n646 = Split 1D Array(array=w1869, index=24) -> (first subarray=→"Labels LSI218 (1)":string[], second subarray=→"Labels LSI218 (2)":string[])
      }
    }
    "LSI218 Status" <- w847
    "error out (LSI218)" <- w830
    n647 = case shown="True" w759 {
      tunnel: [w1759 w1771] -> w817
      tunnel: [w1749 w1770] -> w825
      tunnel: [w1758 w1769] -> w818
      tunnel: [w1757 timestamp[] [] ("TimeArray")] -> w786
      tunnel: [w1756 dbl[][] [] ("DataArray")] -> w784
      tunnel: w827 -> [w1755 w1766]
      tunnel: w826 -> [w1754 w1765]
      tunnel: w767 -> [w1750 _]
      tunnel: w792 -> [_ w1761]
      frame False {
        n648 = local read "Record interval"() -> (w1747:i64)
        n649 = call-dynamic "LSI336Data_measure.vi"("LSI336Data in"=w1755, "MeasurementIndex"=w1750, "error in (no error)"=w1754, "save every ... measurements"=w1747) -> ("Active?"=→"Active?\n(LSI336)":bool[], "TimeMeasuremeent"=→"Time of Last Measurement (LSI336)":timestamp, "LSI336Data out"=w1758:refnum<class "LSI336Data.lvclass">, "LastData"=→"Last Data \nLSI336":dbl[], "LastMeasurementConfig"=→"LastMeasurementConfig (336)":T12, "DataArray"=w1756:dbl[][], "Status"=w1749:u16, "TimeArray"=w1757:timestamp[], "error out"=w1759:errorcluster)  [unwired: 3 in]
      }
      frame True {
        n650 = local read "RUN Identifier"() -> (w1760:string)
        n651 = call-dynamic "LSI336Data_initialize.vi"("LSI336Data in"=w1766, "RunIdentifier"=w1760, "InstName"="InstName (LSI336)", "FileFormat"="FileFormat (336)", "LSI336Settings(X, Y)"="LSI336Settings(X,Y)", "error in (no error)"=w1765, "base path"=w1761) -> ("LSI336Data out"=w1769:refnum<class "LSI336Data.lvclass">, "Status"=w1770:T7, "AllLabels"=→"Labels LSI336":string[], "error out"=w1771:errorcluster)  [unwired: 5 in]
      }
    }
    "LSI336 Status" <- w825
    "error out (LSI336)" <- w817
    "TimeArray (LSI336)" <- w786
    "DataArray (336)" <- w784
    n652 = local read "Last Data \n(USB6210)"() -> (w770:dbl[])
    n653 = local read "Last Data \n(USB6218)"() -> (w771:dbl[])
    n654 = local read "All Labels (USB6210)"() -> (w773:string[])
    n655 = local read "All Labels (USB6218)"() -> (w772:string[])
    n656 = flat-sequence {
      tunnel: w853 -> [w1355]
      tunnel: [w1350] -> w841
      tunnel: [w1348] -> w839
      tunnel: [w1347] -> w836
      tunnel: [w1346] -> w834
      tunnel: w805 -> [w1341]
      frame #0 {
        w1349 = T20 [] ("appended array")
        n657 = Unbundle By Name(w1341) -> ("TimeArray"=w1358:timestamp[], "DataArrayConv"=w1353:dbl[][], "LDArray"=w1352:dbl[])
        n658 = Unbundle By Name(w1355) -> ("ReadLeakDet?"=w1354:bool, "LabelLD"=w1357:string, "Labels"=w1351:string[])  [unwired: 1 out]
        n659 = case shown="True" w1354 {
          tunnel: w1357 -> [_ w1366]
          tunnel: w1353 -> [w1360 w1365]
          tunnel: w1352 -> [_ w1364]
          tunnel: [w1360 w1363] -> w1340
          tunnel: w1351 -> [w1359 w1362]
          tunnel: [w1359 w1361] -> w1343
          frame False {
          }
          frame True {
            n660 = Build Array (concatenate)(w1365, w1364) -> (w1363:dbl[][])
            n661 = Build Array (concatenate)(w1362, w1366) -> (w1361:string[])
          }
        }
        "All Labels (USB6210)" <- w1343
        "DataArrayConv (USB6210)" <- w1340
        n662 = control-ref of="Plot selecter (USB6210)\n    1      2     3     4"() -> (w1342:refnum<vi>)
        n663 = local read "Plot selecter (USB6210)\n    1      2     3     4"() -> (w1345:bool[][])
        n664 = Array Size(array=w1343) -> (size(s)=w1356:i32)
        n665 = Array Size(array=w1343) -> (size(s)=w1344:i32)
        n666 = Array Size(array=w1340) -> (size(s)=→"Data Array sizes (6210)":i32[])
        n667 = property on="Property Node" class="Arr (strict)"(reference=w1342, "Number of Rows"=w1344) -> ()  [unwired: 1 in, 2 out]
        n668 = for {
          N: w1356 -> [_]
          tunnel: w1340 -> [w1387]
          tunnel: w1358 -> [w1388]
          shift-right: [w1383] -> w1348
          shift-left: w1349 -> [w1386]
          shift-right: [w1381] -> w1346
          shift-left: w1349 -> [w1384]
          shift-right: [w1382] -> w1350
          shift-left: w1349 -> [w1380]
          shift-right: [w1379] -> w1347
          shift-left: w1349 -> [w1378]
          tunnel: w1345 -> [w1377]
          i -> [w1372]
          n669 = Index Array(array=w1387, index (col)=w1372) -> (element=w1367:dbl[])  [unwired: 1 in]
          n670 = Index Array(array=w1377, index (row) #1=w1372, index (col) #1=0 ("index (row)"), index (row) #2=w1372, index (col) #2=1 ("index (row)"), index (row) #3=w1372, index (col) #3=2 ("index (row)"), index (row) #4=w1372, index (col) #4=3 ("index (row)")) -> (element #1=w1371:bool, element #2=w1370:bool, element #3=w1369:bool, element #4=w1368:bool)
          n671 = Bundle("TimeArray"=w1388, "DataArrayConv"=w1367) -> (w1385:T23)  [unwired: 1 in]
          n672 = stacked-sequence {
            tunnel: w1371 -> [w1392 _ _ _]
            tunnel: w1386 -> [_ w1400 _ _]
            tunnel: w1369 -> [_ _ w1408 _]
            tunnel: w1385 -> [w1389 w1398 w1407 w1413]
            tunnel: w1368 -> [_ _ _ w1416]
            tunnel: w1384 -> [_ _ _ w1415]
            tunnel: [_ _ _ w1414] -> w1381
            tunnel: [_ w1399 _ _] -> w1383
            tunnel: [w1391 _ _ _] -> w1382
            tunnel: w1380 -> [w1390 _ _ _]
            tunnel: [_ _ w1406 _] -> w1379
            tunnel: w1378 -> [_ _ w1405 _]
            tunnel: w1370 -> [_ w1397 _ _]
            frame #0 {
              n673 = case shown="True" w1392 {
                tunnel: [w1393 w1396] -> w1391
                tunnel: w1389 -> [_ w1395]
                tunnel: w1390 -> [w1393 w1394]
                frame False {
                }
                frame True {
                  n674 = Build Array (concatenate)(w1394, w1395) -> (w1396:T20)
                }
              }
            }
            frame #1 {
              n675 = case shown="True" w1397 {
                tunnel: w1400 -> [w1401 w1404]
                tunnel: [w1401 w1403] -> w1399
                tunnel: w1398 -> [_ w1402]
                frame False {
                }
                frame True {
                  n676 = Build Array (concatenate)(w1404, w1402) -> (w1403:T20)
                }
              }
            }
            frame #2 {
              n677 = case shown="True" w1408 {
                tunnel: [w1409 w1412] -> w1406
                tunnel: w1407 -> [_ w1411]
                tunnel: w1405 -> [w1409 w1410]
                frame False {
                }
                frame True {
                  n678 = Build Array (concatenate)(w1410, w1411) -> (w1412:T20)
                }
              }
            }
            frame #3 {
              n679 = case shown="True" w1416 {
                tunnel: [w1417 w1420] -> w1414
                tunnel: w1413 -> [_ w1419]
                tunnel: w1415 -> [w1417 w1418]
                frame False {
                }
                frame True {
                  n680 = Build Array (concatenate)(w1418, w1419) -> (w1420:T20)
                }
              }
            }
          }
        }
      }
    }
    n681 = case shown="True" "Digital Out ON?" {
      tunnel: w759 -> [_ w1478]
      tunnel: w807 -> [w1471 w1477]
      tunnel: [w1471 w1476] -> w806
      tunnel: w805 -> [_ w1475]
      tunnel: w760 -> [_ w1474]
      tunnel: w792 -> [_ w1473]
      tunnel: w787 -> [_ w1472]
      frame False {
      }
      frame True {
        n682 = case shown="False" w1478 {
          tunnel: w1477 -> [w1493 w1653]
          tunnel: [w1493 w1674] -> w1476
          tunnel: w1475 -> [w1494 _]
          tunnel: w1474 -> [_ w1662]
          tunnel: w1473 -> [_ w1645]
          tunnel: w1472 -> [_ _]
          frame False {
            n683 = flat-sequence {
              frame #0 {
              }
            }
            n684 = local read "All Labels (USB6210)"() -> (w1482:string[])
            n685 = Multiply(x="N for sampling", y=i64 2) -> (x*y=w1488:i64)
            n686 = local read "Cycle #"() -> (w1492:u32)
            n687 = Search 1D Array(1D array=w1482, element="Auto Fll\nDewar P. label") -> (index of element=→"Target Index (P)":i32)  [unwired: 1 in]
            n688 = Search 1D Array(1D array=w1482, element="Auto Fll\nHe level label") -> (index of element=→"Target Index (L)":i32)  [unwired: 1 in]
            n689 = Add(x=w1488, y="Mov. Avg Interval") -> (x+y=w1490:i64)
            n690 = Greater?(x=w1492, y=w1490) -> (0:w1486:bool)
            n691 = And(x=w1486, y="Auto Fill ON?") -> (x .and. y?=w1484:bool)
            n692 = case shown="True" w1484 {
              tunnel: w1494 -> [_ w1525]
              tunnel: "Mov. Avg Interval" -> [_ w1509]
              tunnel: w1488 -> [_ w1495]
              tunnel: "N for sampling" -> [_ w1507]
              frame False {
              }
              frame True {
                n693 = local read "Pstd"() -> (→"Pstd history":dbl)
                n694 = local read "Lstd"() -> (→"Lstd history":dbl)
                n695 = local read "Pav (Pa)"() -> (→"Pav history":dbl)
                n696 = local read "Lav (%)"() -> (→"Lav history":dbl)
                n697 = local read "Target Index (P)"() -> (w1526:i32)
                n698 = local read "Target Index (L)"() -> (w1512:i32)
                n699 = Unbundle By Name(w1525) -> ("TimeArray"=w1523:timestamp[], "DataArrayConv"=w1524:dbl[][])
                n700 = Index Array(array=w1524, index (col) #1=w1526, index (col) #2=w1512) -> (element #1=w1511:dbl[], element #2=w1506:dbl[])  [unwired: 2 in]
                n701 = Delete From Array(array=w1511, length=w1495) -> (deleted portion=w1520:dbl[])  [unwired: 1 in, 1 out]
                n702 = Delete From Array(array=w1506, length=w1495) -> (deleted portion=w1505:dbl[])  [unwired: 1 in, 1 out]
                n703 = call "MovingAverage.vi"("Moving Average interval"=w1509, "Input Array"=w1506) -> ("M.A. Array"=w1508:dbl[])  [unwired: 9 in]
                n704 = call "MovingAverage.vi"("Moving Average interval"=w1509, "Input Array"=w1511) -> ("M.A. Array"=w1510:dbl[])  [unwired: 9 in]
                n705 = Delete From Array(array=w1510, length=w1495) -> (deleted portion=w1521:dbl[])  [unwired: 1 in, 1 out]
                n706 = Delete From Array(array=w1510, length=w1495) -> (deleted portion=w1517:dbl[])  [unwired: 1 in, 1 out]
                "Last N M.A. Pressures" <- w1517
                n707 = Delete From Array(array=w1508, length=w1495) -> (deleted portion=w1500:dbl[])  [unwired: 1 in, 1 out]
                "Last N M.A. Levels" <- w1500
                n708 = Delete From Array(array=w1523, length=w1495) -> (deleted portion=w1502:timestamp[])  [unwired: 1 in, 1 out]
                n709 = Bundle("TimeArray"=w1502, "DataArrayConv"=w1520) -> (w1519:T23)  [unwired: 1 in]
                n710 = Bundle("TimeArray"=w1502, "M.A. Array"=w1521) -> (w1522:T24)  [unwired: 1 in]
                n711 = Bundle("TimeArray"=w1502, "DataArrayConv"=w1505) -> (w1504:T23)  [unwired: 1 in]
                n712 = Bundle("TimeArray"=w1502, "M.A. Array"=w1500) -> (w1501:T24)  [unwired: 1 in]
                n713 = Array Size(array=w1517) -> (size(s)=w1516:i32)
                n714 = Greater Or Equal?(x=w1516, y=w1507) -> (x >= y?=w1515:bool)
                n715 = Build Array(w1519, w1522) -> (→"Dewar Pressure":T25)
                n716 = Build Array(w1504, w1501) -> (→"He Level":T25)
                n717 = case shown="True" w1515 {
                  tunnel: [w1630 w1635] -> w1499
                  tunnel: w1517 -> [_ w1636]
                  tunnel: w1500 -> [_ w1633]
                  tunnel: [w1630 w1631] -> w1498
                  frame False {
                    w1630 = nan ("mean")
                  }
                  frame True {
                    n718 = call <vilib>:"Std Deviation and Variance.vi"("X"=w1636) -> ("mean"=w1635:dbl, "standard deviation"=w1634:dbl)  [unwired: 1 in, 1 out]
                    n719 = call <vilib>:"Std Deviation and Variance.vi"("X"=w1633) -> ("mean"=w1631:dbl, "standard deviation"=w1632:dbl)  [unwired: 1 in, 1 out]
                    n720 = local write "Pstd"(w1634) -> ()
                    n721 = local write "Lstd"(w1632) -> ()
                    n722 = local write "Pav (Pa)"(w1635) -> ()
                    n723 = local write "Lav (%)"(w1631) -> ()
                  }
                }
                n724 = flat-sequence {
                  tunnel: w1499 -> [w1527]
                  tunnel: w1498 -> [w1528]